vi "Tester_v01.vi"() -> ()   [LabVIEW 2015]
uses:
  <vilib>/LabVIEW Interface for Arduino/Type Defs/Pin Mode.ctl
  <vilib>/LabVIEW Interface for Arduino/LabVIEW Interface for Arduino.lvlib
panel:
  out "Test pass 2":string
  out "Welcome Message":string
  out "K4 voltage":dbl(knob) scale=0.0..5.0
  out "J16":dbl(knob) scale=0.0..5.0
  out "K3 voltage 2":dbl(knob) scale=0.0..5.0
  out "J6":dbl(knob) scale=0.0..5.0
  out "K2 voltage":dbl(knob) scale=0.0..5.0
  out "K1 voltage":dbl(knob) scale=0.0..5.0
  out "Tab Control":T1(tab)
  out "Please wait":string
  in  "Exit the program":bool
  in  "Start Test":bool
  in  "CONTINUE 2":bool
  out "Message Page 2":string
  in  "START page 3":bool
  out "Wire connection 3":string
  in  "NO LED ON":bool
  in  "YES LED ON":bool
  out "LED ON?":string
  out "Error message":string
  in  "STOP K1 LED ON":bool
  out "LED OFF?":string
  in  "YES LED OFF":bool
  in  "NO LED OFF":bool
  in  "STOP K1 LED OFF":bool
  out "Loading bar":string
  out "Progress Bar":u8(slide) scale=0.0..100.0
  in  "Stop K1":bool
  in  "STOP K2":bool
  in  "STOP K3":bool
  in  "STOP K4":bool
  in  "STOPJ6":bool
  in  "STOP J16":bool
  in  "STOP J4 error":bool
  out "Test pass":string
  in  "Complete":bool
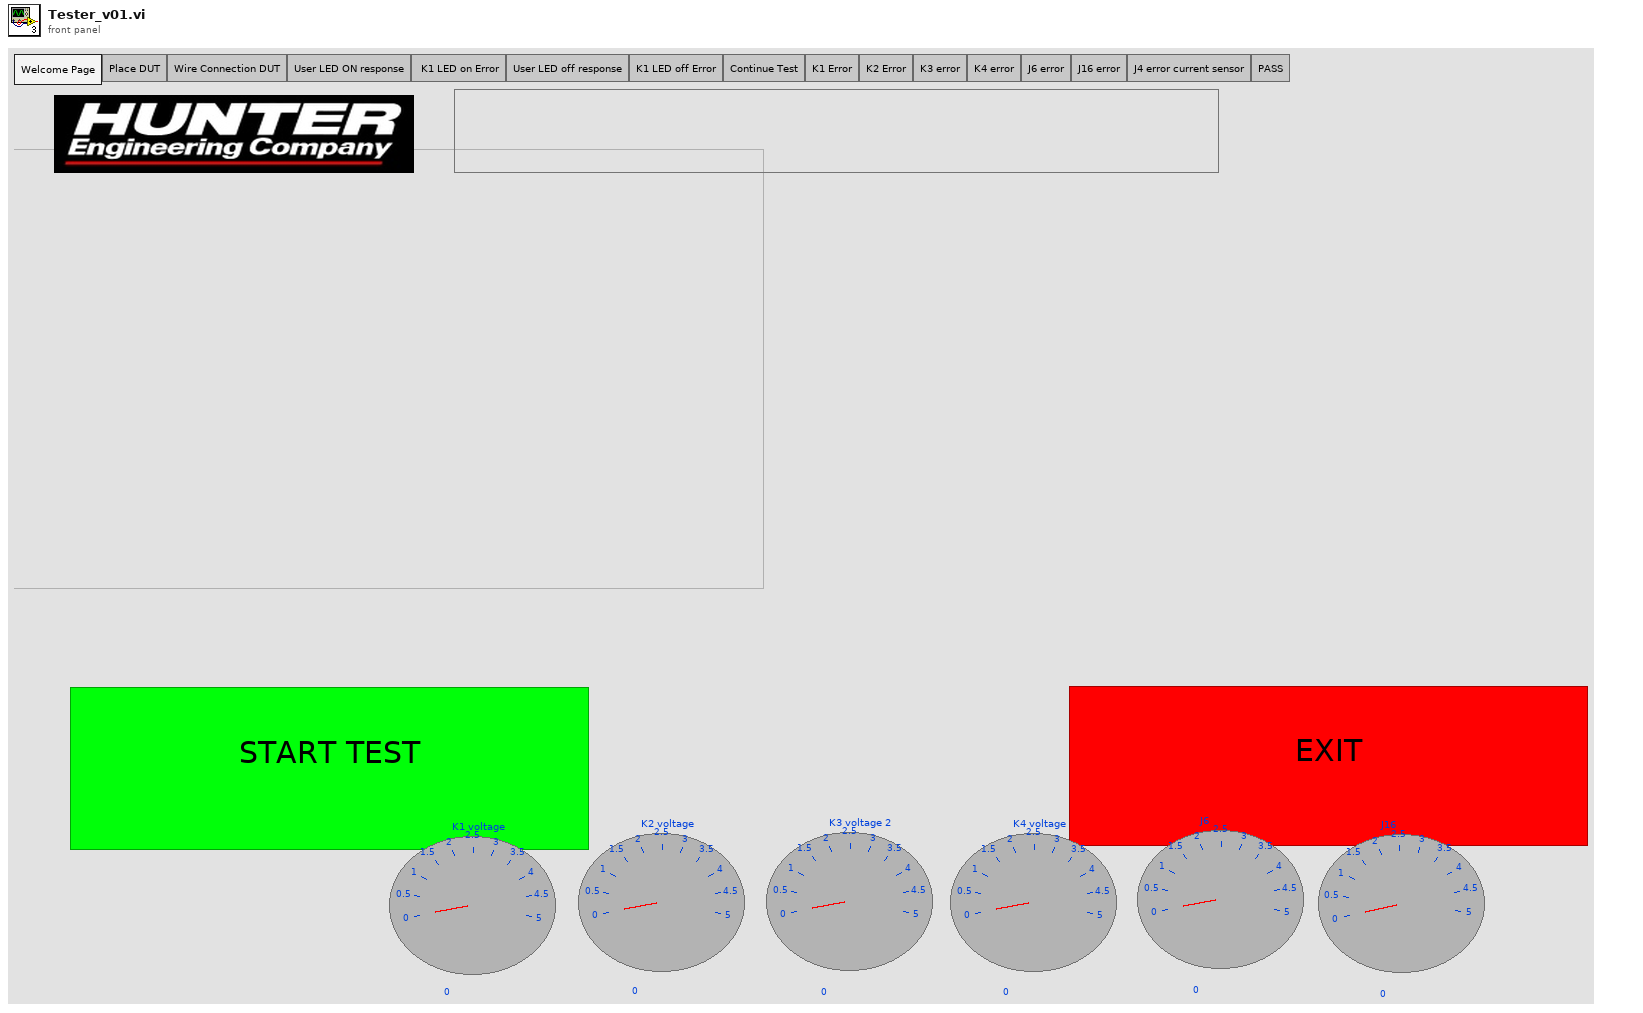
[diagram p1: front panel]
types:
  T1 = enum32{"Welcome Page", "Place DUT", "Wire Connection DUT", "User LED ON response", " K1 LED on Error", "User LED off response", "K1 LED off Error", "Continue Test", "K1 Error", "K2 Error", "K3 error", "K4 error", "J6 error", "J16 error", "J4 error current sensor", "PASS"}
  T2 = typedef "LabVIEW Interface for Arduino.lvlib/Pin Mode.ctl" = enum8{"Input", "Output"}
  T3 = enum8{"Enabled", "Disabled", "Disabled and Grayed Out"}
  T4 = typedef "LabVIEW Interface for Arduino.lvlib/Arduino Resource.ctl" = cluster{"VISA resource":refnum<visa-resource-name>, "Board Type":T5, "Connection Type":enum8{"USB / Serial"}, "Bytes Per Packet (15)":u8}
  T5 = typedef "LabVIEW Interface for Arduino.lvlib/Board Type.ctl" = enum16{"Uno", "Dimuelanove w/Atmega 328", "Mega 2560"}
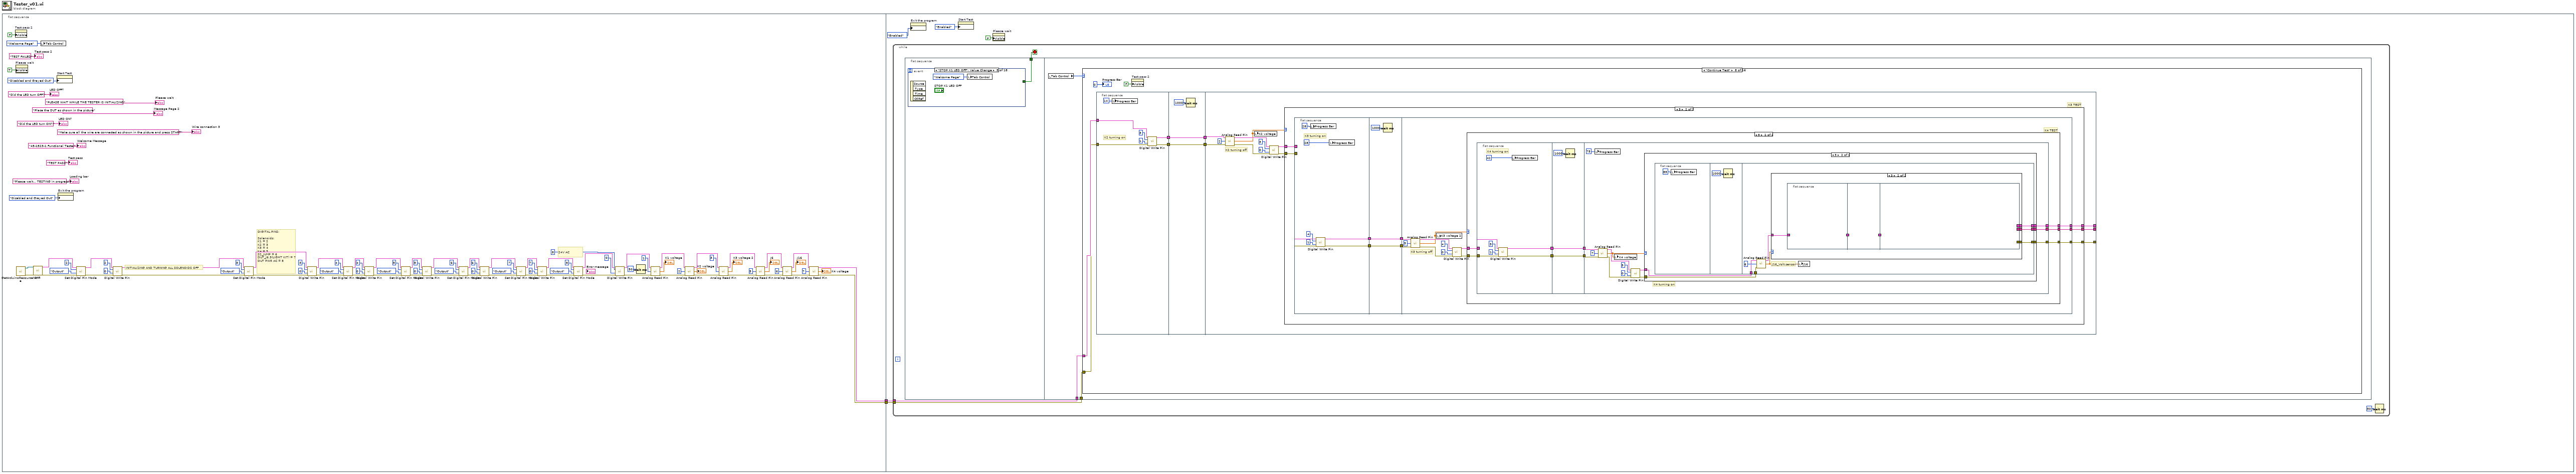
[diagram p0: block diagram]
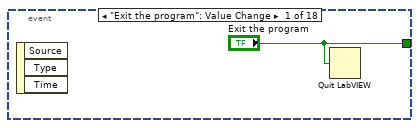
[diagram p2: hidden frame]
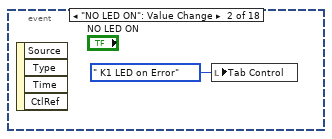
[diagram p3: hidden frame]
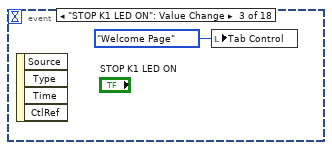
[diagram p4: hidden frame]
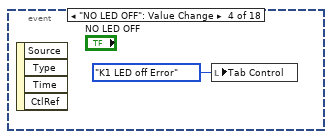
[diagram p5: hidden frame]
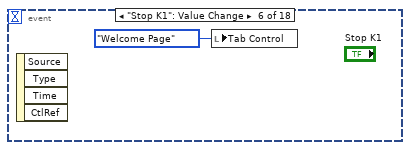
[diagram p6: hidden frame]
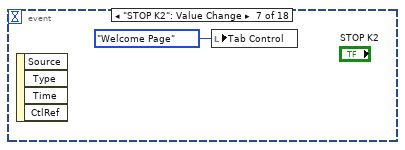
[diagram p7: hidden frame]
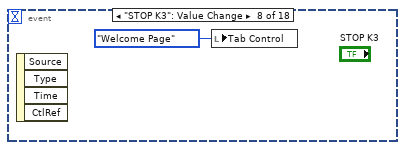
[diagram p8: hidden frame]
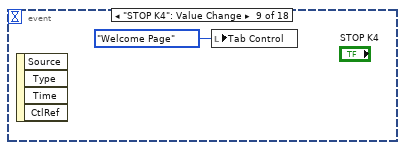
[diagram p9: hidden frame]
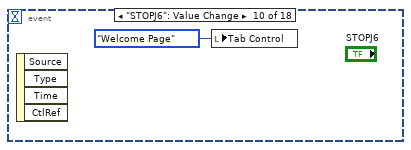
[diagram p10: hidden frame]
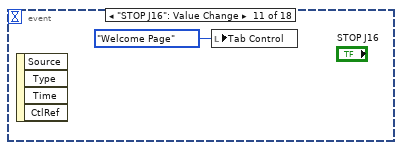
[diagram p11: hidden frame]
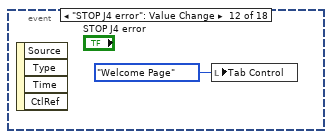
[diagram p12: hidden frame]
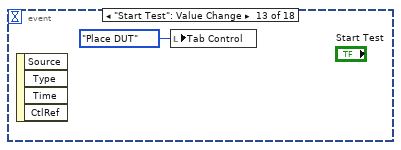
[diagram p13: hidden frame]
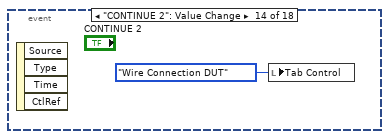
[diagram p14: hidden frame]
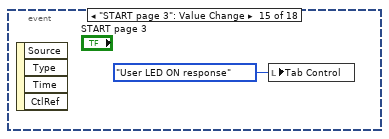
[diagram p15: hidden frame]
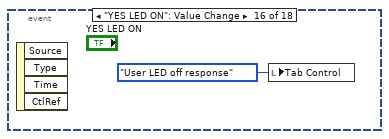
[diagram p16: hidden frame]
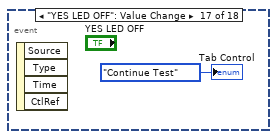
[diagram p17: hidden frame]
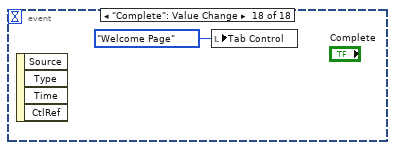
[diagram p18: hidden frame]
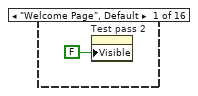
[diagram p19: hidden frame]
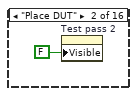
[diagram p20: hidden frame]
diagram:
  n1 = flat-sequence {
    tunnel: [w6] -> w2
    tunnel: [w5] -> w1
    tunnel: w2 -> [w106]
    tunnel: w1 -> [w105]
    frame #0 {
      # "24V AC"
      # "DIGITAL PINS:\n\nSolenoids:\nK1 = 2\nK2 = 3\nK3 = 4\nK4 = 5\nS2_JUMP = 6\nDUT_J6.3(LIGHT KIT) = 7\nDUT PWR AC = 8"
      # "INITIALIZING AND TURNING ALL SOLENOIDS OFF"
      n2 = property on="Test pass 2" class="Str"("Visible"=FALSE) -> ()  [unwired: 2 in, 2 out]
      n3 = property on="Please wait" class="Str"("Visible"=TRUE) -> ()  [unwired: 2 in, 2 out]
      n4 = call "GetArduinoResourceName.vi"() -> ("error out"=w39:errorcluster, "VISA resource name"=w40:refnum<visa-resource-name>)  [unwired: 10 in]
      n5 = call <vilib>:"Init.vi"("VISA resource"=w40, "error in"=w39) -> ("Arduino Resource"=w76:T4, "error out"=w75:errorcluster)  [unwired: 16 in]
      n6 = local write "Tab Control"(T1."Welcome Page" ("Tab Control")) -> ()
      n7 = property on="Start Test" class="Bool (strict)"("DisabledEnum"=T3."Disabled and Grayed Out" ("Disabled")) -> ()  [unwired: 2 in, 2 out]
      n8 = property on="Exit the program" class="Bool (strict)"("DisabledEnum"=T3."Disabled and Grayed Out" ("Disabled")) -> ()  [unwired: 2 in, 2 out]
      n9 = call <vilib>:"Set Digital Pin Mode.vi"("Arduino Resource"=w76, "Digital I/O Pin"=u8 2, "Pin Mode (Input)"=Pin_Mode."Output", "error in"=w75) -> ("Arduino Resource"=w96:T4, "error out"=w97:errorcluster)  [unwired: 10 in]
      n10 = call <vilib>:"Digital Write Pin.vi"("Arduino Resource"=w96, "Digital I/O Pin (0)"=u8 2 ("Digital I/O Pin"), "Value (0)"=u8 0, "error in"=w97) -> ("Arduino Resource"=w88:T4, "error out"=w87:errorcluster)  [unwired: 10 in]
      n11 = call <vilib>:"Set Digital Pin Mode.vi"("Arduino Resource"=w88, "Digital I/O Pin"=u8 3, "Pin Mode (Input)"=Pin_Mode."Output", "error in"=w87) -> ("Arduino Resource"=w91:T4, "error out"=w90:errorcluster)  [unwired: 10 in]
      n12 = call <vilib>:"Digital Write Pin.vi"("Arduino Resource"=w91, "Digital I/O Pin (0)"=u8 3 ("Digital I/O Pin"), "Value (0)"=u8 0, "error in"=w90) -> ("Arduino Resource"=w78:T4, "error out"=w77:errorcluster)  [unwired: 10 in]
      n13 = call <vilib>:"Set Digital Pin Mode.vi"("Arduino Resource"=w78, "Digital I/O Pin"=u8 4, "Pin Mode (Input)"=Pin_Mode."Output", "error in"=w77) -> ("Arduino Resource"=w42:T4, "error out"=w80:errorcluster)  [unwired: 10 in]
      n14 = call <vilib>:"Digital Write Pin.vi"("Arduino Resource"=w42, "Digital I/O Pin (0)"=u8 4 ("Digital I/O Pin"), "Value (0)"=u8 0, "error in"=w80) -> ("Arduino Resource"=w85:T4, "error out"=w86:errorcluster)  [unwired: 10 in]
      n15 = call <vilib>:"Set Digital Pin Mode.vi"("Arduino Resource"=w85, "Digital I/O Pin"=u8 5, "Pin Mode (Input)"=Pin_Mode."Output", "error in"=w86) -> ("Arduino Resource"=w36:T4, "error out"=w24:errorcluster)  [unwired: 10 in]
      n16 = call <vilib>:"Digital Write Pin.vi"("Arduino Resource"=w36, "Digital I/O Pin (0)"=u8 5 ("Digital I/O Pin"), "Value (0)"=u8 0, "error in"=w24) -> ("Arduino Resource"=w48:T4, "error out"=w47:errorcluster)  [unwired: 10 in]
      n17 = call <vilib>:"Set Digital Pin Mode.vi"("Arduino Resource"=w48, "Digital I/O Pin"=u8 6, "Pin Mode (Input)"=Pin_Mode."Output", "error in"=w47) -> ("Arduino Resource"=w55:T4, "error out"=w67:errorcluster)  [unwired: 10 in]
      n18 = call <vilib>:"Digital Write Pin.vi"("Arduino Resource"=w55, "Digital I/O Pin (0)"=u8 6 ("Digital I/O Pin"), "Value (0)"=u8 0, "error in"=w67) -> ("Arduino Resource"=w52:T4, "error out"=w51:errorcluster)  [unwired: 10 in]
      n19 = call <vilib>:"Set Digital Pin Mode.vi"("Arduino Resource"=w52, "Digital I/O Pin"=u8 7, "Pin Mode (Input)"=Pin_Mode."Output", "error in"=w51) -> ("Arduino Resource"=w54:T4, "error out"=w64:errorcluster)  [unwired: 10 in]
      n20 = call <vilib>:"Digital Write Pin.vi"("Arduino Resource"=w54, "Digital I/O Pin (0)"=u8 7 ("Digital I/O Pin"), "Value (0)"=u8 0, "error in"=w64) -> ("Arduino Resource"=w50:T4, "error out"=w49:errorcluster)  [unwired: 10 in]
      n21 = call <vilib>:"Set Digital Pin Mode.vi"("Arduino Resource"=w50, "Digital I/O Pin"=u8 8, "Pin Mode (Input)"=Pin_Mode."Output", "error in"=w49) -> ("Arduino Resource"=w53:T4, "error out"=w57:errorcluster)  [unwired: 10 in]
      n22 = call <vilib>:"Digital Write Pin.vi"("Arduino Resource"=w53, "Digital I/O Pin (0)"=u8 8 ("Digital I/O Pin"), "Value (0)"=u8 0, "error in"=w57) -> ("Arduino Resource"=w13:T4, "error out"=w14:errorcluster)  [unwired: 10 in]
      n23 = Wait (ms)(milliseconds to wait=u32 50) -> ()  [unwired: 1 out]
      n24 = call <vilib>:"Analog Read Pin.vi"("Arduino Resource"=w13, "Analog Input Pin (0)"=u8 1, "error in"=w14) -> ("Arduino Resource"=w4:T4, "Voltage"=→"K1 voltage":dbl, "error out"=w25:errorcluster)  [unwired: 10 in]
      n25 = call <vilib>:"Analog Read Pin.vi"("Arduino Resource"=w4, "Analog Input Pin (0)"=u8 2, "error in"=w25) -> ("Arduino Resource"=w3:T4, "Voltage"=→"K2 voltage":dbl, "error out"=w20:errorcluster)  [unwired: 10 in]
      n26 = call <vilib>:"Analog Read Pin.vi"("Arduino Resource"=w3, "Analog Input Pin (0)"=u8 3, "error in"=w20) -> ("Arduino Resource"=w23:T4, "Voltage"=→"K3 voltage 2":dbl, "error out"=w21:errorcluster)  [unwired: 10 in]
      n27 = call <vilib>:"Analog Read Pin.vi"("Arduino Resource"=w23, "Analog Input Pin (0)"=u8 5, "error in"=w21) -> ("Arduino Resource"=w22:T4, "Voltage"=→"J6":dbl, "error out"=w19:errorcluster)  [unwired: 10 in]
      n28 = call <vilib>:"Analog Read Pin.vi"("Arduino Resource"=w22, "Analog Input Pin (0)"=u8 6, "error in"=w19) -> ("Arduino Resource"=w16:T4, "Voltage"=→"J16":dbl, "error out"=w17:errorcluster)  [unwired: 10 in]
      n29 = call <vilib>:"Analog Read Pin.vi"("Arduino Resource"=w16, "Analog Input Pin (0)"=u8 7, "error in"=w17) -> ("Arduino Resource"=w6:T4, "Voltage"=→"K4 voltage":dbl, "error out"=w5:errorcluster)  [unwired: 10 in]
      "Welcome Message" <- "45-1523-1 Functional Tester"
      "Message Page 2" <- "Place the DUT as shown in the picture"
      "Wire connection 3" <- "Make sure all the wire are connected as shown in the picture and press START" ("Wire connection 3")
      "LED ON?" <- "Did the LED turn ON?!" ("LED ON?")
      "LED OFF?" <- "Did the LED turn OFF?" ("LED OFF?")
      "Loading bar" <- "Please wait... TESTING in progress" ("Loading bar")
      "Test pass" <- "TEST PASS" ("Test pass")
      "Please wait" <- "PLEASE WAIT WHILE THE TESTER IS INITIALIZING" ("Please wait")
      "Test pass 2" <- "TEST FAILED" ("Test pass 2")
    }
    frame #1 {
      n30 = while {
        tunnel: w106 -> [w109]
        tunnel: w105 -> [w108]
        stop <- w107 stop-if-true
        n31 = flat-sequence {
          tunnel: [w111] -> w107
          tunnel: w109 -> [w132]
          tunnel: w108 -> [w131]
          frame #0 {
            n32 = event shown="[4] \"STOP K1 LED OFF\": Value Change" {
              selector: _ -> [_ _ _ _ _ _ _ _ _ _ _ _ _ _ _ _ _ _]
              dyn-events: _ -> [_ _ _ _ _ _ _ _ _ _ _ _ _ _ _ _ _ _]
              timeout: _ -> [_ _ _ _ _ _ _ _ _ _ _ _ _ _ _ _ _ _]
              tunnel: ["Exit the program" _ _ _ _ _ _ _ _ _ _ _ _ _ _ _ _ _] -> w111
              event "Exit the program": Value Change {
                n33 = event-data() -> ()  [unwired: 1 in, 3 out]
                n34 = Quit LabVIEW(quit? (T)="Exit the program") -> ()
              }
              event "NO LED ON": Value Change {
                n35 = event-data() -> ()  [unwired: 1 in, 4 out]
                n36 = local write "Tab Control"(T1." K1 LED on Error" ("Tab Control")) -> ()
              }
              event "STOP K1 LED ON": Value Change {
                n37 = event-data() -> ()  [unwired: 1 in, 4 out]
                n38 = local write "Tab Control"(T1."Welcome Page" ("Tab Control")) -> ()
              }
              event "NO LED OFF": Value Change {
                n39 = event-data() -> ()  [unwired: 1 in, 4 out]
                n40 = local write "Tab Control"(T1."K1 LED off Error" ("Tab Control")) -> ()
              }
              event "STOP K1 LED OFF": Value Change {
                n41 = event-data() -> ()  [unwired: 1 in, 4 out]
                n42 = local write "Tab Control"(T1."Welcome Page" ("Tab Control")) -> ()
              }
              event "Stop K1": Value Change {
                n43 = event-data() -> ()  [unwired: 1 in, 4 out]
                n44 = local write "Tab Control"(T1."Welcome Page" ("Tab Control")) -> ()
              }
              event "STOP K2": Value Change {
                n45 = event-data() -> ()  [unwired: 1 in, 4 out]
                n46 = local write "Tab Control"(T1."Welcome Page" ("Tab Control")) -> ()
              }
              event "STOP K3": Value Change {
                n47 = event-data() -> ()  [unwired: 1 in, 4 out]
                n48 = local write "Tab Control"(T1."Welcome Page" ("Tab Control")) -> ()
              }
              event "STOP K4": Value Change {
                n49 = event-data() -> ()  [unwired: 1 in, 4 out]
                n50 = local write "Tab Control"(T1."Welcome Page" ("Tab Control")) -> ()
              }
              event "STOPJ6": Value Change {
                n51 = event-data() -> ()  [unwired: 1 in, 4 out]
                n52 = local write "Tab Control"(T1."Welcome Page" ("Tab Control")) -> ()
              }
              event "STOP J16": Value Change {
                n53 = event-data() -> ()  [unwired: 1 in, 4 out]
                n54 = local write "Tab Control"(T1."Welcome Page" ("Tab Control")) -> ()
              }
              event "STOP J4 error": Value Change {
                n55 = event-data() -> ()  [unwired: 1 in, 4 out]
                n56 = local write "Tab Control"(T1."Welcome Page" ("Tab Control")) -> ()
              }
              event "Start Test": Value Change {
                n57 = event-data() -> ()  [unwired: 1 in, 4 out]
                n58 = local write "Tab Control"(T1."Place DUT" ("Tab Control")) -> ()
              }
              event "CONTINUE 2": Value Change {
                n59 = event-data() -> ()  [unwired: 1 in, 4 out]
                n60 = local write "Tab Control"(T1."Wire Connection DUT" ("Tab Control")) -> ()
              }
              event "START page 3": Value Change {
                n61 = event-data() -> ()  [unwired: 1 in, 4 out]
                n62 = local write "Tab Control"(T1."User LED ON response" ("Tab Control")) -> ()
              }
              event "YES LED ON": Value Change {
                n63 = event-data() -> ()  [unwired: 1 in, 4 out]
                n64 = local write "Tab Control"(T1."User LED off response" ("Tab Control")) -> ()
              }
              event "YES LED OFF": Value Change {
                n65 = event-data() -> ()  [unwired: 1 in, 4 out]
                "Tab Control" <- T1."Continue Test" ("Tab Control")
              }
              event "Complete": Value Change {
                n66 = event-data() -> ()  [unwired: 1 in, 4 out]
                n67 = local write "Tab Control"(T1."Welcome Page" ("Tab Control")) -> ()
              }
            }
          }
          frame #1 {
            n68 = local read "Tab Control"() -> (w130:T1)
            n69 = case shown="\"Continue Test\"" w130 {
              tunnel: w132 -> [_ _ _ w149 _ w186 _ w210 _ _ _ _ _ _ _ _]
              tunnel: w131 -> [_ _ _ w148 _ w185 _ w209 _ _ _ _ _ _ _ _]
              frame "Welcome Page", Default {
                n70 = property on="Test pass 2" class="Str"("Visible"=FALSE) -> ()  [unwired: 2 in, 2 out]
              }
              frame "Place DUT" {
                n71 = property on="Test pass 2" class="Str"("Visible"=FALSE) -> ()  [unwired: 2 in, 2 out]
              }
              frame "Wire Connection DUT" {
                n72 = property on="Test pass 2" class="Str"("Visible"=FALSE) -> ()  [unwired: 2 in, 2 out]
              }
              frame "User LED ON response" {
                n73 = flat-sequence {
                  tunnel: w149 -> [w153]
                  tunnel: w148 -> [w152]
                  tunnel: [w151] -> w139
                  tunnel: [w150] -> w137
                  tunnel: w139 -> [w158]
                  tunnel: [w158] -> w138
                  tunnel: w137 -> [w157]
                  tunnel: [w157] -> w136
                  tunnel: w138 -> [w163]
                  tunnel: [w162] -> w141
                  tunnel: [w161] -> w140
                  tunnel: w136 -> [w160]
                  tunnel: [w166] -> w147
                  tunnel: [w165] -> w146
                  tunnel: w141 -> [w166]
                  tunnel: w140 -> [w165]
                  tunnel: w147 -> [w172]
                  tunnel: w146 -> [w171]
                  tunnel: [w170] -> w144
                  tunnel: [w169] -> w143
                  tunnel: [w168] -> w142
                  tunnel: w144 -> [w177]
                  tunnel: w143 -> [w176]
                  tunnel: w142 -> [w178]
                  frame #0 {
                    n74 = call <vilib>:"Digital Write Pin.vi"("Arduino Resource"=w153, "Digital I/O Pin (0)"=u8 8, "Value (0)"=u8 1, "error in"=w152) -> ("Arduino Resource"=w150:T4, "error out"=w151:errorcluster)  [unwired: 10 in]
                  }
                  frame #1 {
                    n75 = Wait (ms)(milliseconds to wait=u32 1000) -> ()  [unwired: 1 out]
                  }
                  frame #2 {
                    n76 = call <vilib>:"Digital Write Pin.vi"("Arduino Resource"=w160, "Digital I/O Pin (0)"=u8 2, "Value (0)"=u8 1, "error in"=w163) -> ("Arduino Resource"=w162:T4, "error out"=w161:errorcluster)  [unwired: 10 in]
                  }
                  frame #3 {
                    n77 = Wait (ms)(milliseconds to wait=u32 1000) -> ()  [unwired: 1 out]
                  }
                  frame #4 {
                    n78 = call <vilib>:"Analog Read Pin.vi"("Arduino Resource"=w172, "Analog Input Pin (0)"=u8 1, "error in"=w171) -> ("Arduino Resource"=w168:T4, "Voltage"=w169:dbl, "error out"=w170:errorcluster)  [unwired: 10 in]
                  }
                  frame #5 {
                    n79 = call <vilib>:"Digital Write Pin.vi"("Arduino Resource"=w178, "Digital I/O Pin (0)"=u8 2, "Value (0)"=u8 0, "error in"=w177) -> ()  [unwired: 10 in, 2 out]
                    n80 = local write "K1 voltage"(w176) -> ()
                  }
                }
                n81 = property on="Test pass 2" class="Str"("Visible"=FALSE) -> ()  [unwired: 2 in, 2 out]
              }
              frame " K1 LED on Error" {
                n82 = property on="Test pass 2" class="Str"("Visible"=TRUE) -> ()  [unwired: 2 in, 2 out]
              }
              frame "User LED off response" {
                n83 = flat-sequence {
                  tunnel: w186 -> [w194]
                  tunnel: w185 -> [w193]
                  tunnel: [w189] -> w183
                  tunnel: [w188] -> w181
                  tunnel: [w198] -> w184
                  tunnel: w183 -> [w198]
                  tunnel: [w197] -> w182
                  tunnel: w181 -> [w197]
                  tunnel: w184 -> [w202]
                  tunnel: w182 -> [w201]
                  frame #0 {
                    n84 = call <vilib>:"Digital Write Pin.vi"("Arduino Resource"=w194, "Digital I/O Pin (0)"=u8 7, "Value (0)"=u8 1, "error in"=w193) -> ("Arduino Resource"=w191:T4, "error out"=w190:errorcluster)  [unwired: 10 in]
                    n85 = call <vilib>:"Digital Write Pin.vi"("Arduino Resource"=w191, "Digital I/O Pin (0)"=u8 6, "Value (0)"=u8 1, "error in"=w190) -> ("Arduino Resource"=w189:T4, "error out"=w188:errorcluster)  [unwired: 10 in]
                  }
                  frame #1 {
                    n86 = Wait (ms)(milliseconds to wait=u32 250) -> ()  [unwired: 1 out]
                  }
                  frame #2 {
                    n87 = call <vilib>:"Digital Write Pin.vi"("Arduino Resource"=w202, "Digital I/O Pin (0)"=u8 7, "Value (0)"=u8 0, "error in"=w201) -> ("Arduino Resource"=w206:T4, "error out"=w207:errorcluster)  [unwired: 10 in]
                    n88 = call <vilib>:"Digital Write Pin.vi"("Arduino Resource"=w206, "Digital I/O Pin (0)"=u8 6, "Value (0)"=u8 0, "error in"=w207) -> ()  [unwired: 10 in, 2 out]
                  }
                }
                n89 = property on="Test pass 2" class="Str"("Visible"=FALSE) -> ()  [unwired: 2 in, 2 out]
              }
              frame "K1 LED off Error" {
                n90 = property on="Test pass 2" class="Str"("Visible"=TRUE) -> ()  [unwired: 2 in, 2 out]
              }
              frame "Continue Test" {
                n91 = flat-sequence {
                  tunnel: [w221] -> w215
                  tunnel: [w220] -> w214
                  tunnel: w210 -> [w218]
                  tunnel: w209 -> [w217]
                  tunnel: w215 -> [w224]
                  tunnel: [w225] -> w213
                  tunnel: w214 -> [w225]
                  tunnel: [w224] -> w212
                  tunnel: w213 -> [w238]
                  tunnel: w212 -> [w237]
                  tunnel: [w230] -> _
                  tunnel: [w228] -> _
                  tunnel: [w227] -> _
                  frame #0 {
                    # "K2 turning on"
                    n92 = local write "Progress Bar"(u8 14 ("Progress Bar")) -> ()
                    n93 = call <vilib>:"Digital Write Pin.vi"("Arduino Resource"=w218, "Digital I/O Pin (0)"=u8 3, "Value (0)"=u8 1, "error in"=w217) -> ("Arduino Resource"=w221:T4, "error out"=w220:errorcluster)  [unwired: 10 in]
                  }
                  frame #1 {
                    n94 = Wait (ms)(milliseconds to wait=u32 1000) -> ()  [unwired: 1 out]
                  }
                  frame #2 {
                    # "K3 TEST"
                    # "K2 turning off"
                    n95 = call <vilib>:"Analog Read Pin.vi"("Arduino Resource"=w237, "Analog Input Pin (0)"=u8 2, "error in"=w238) -> ("Arduino Resource"=w236:T4, "Voltage"=w229:dbl, "error out"=w235:errorcluster)  [unwired: 10 in]
                    n96 = local write "K2 voltage"(w229) -> ()
                    n97 = call <vilib>:"Digital Write Pin.vi"("Arduino Resource"=w236, "Digital I/O Pin (0)"=u8 3, "Value (0)"=u8 0, "error in"=w235) -> ("Arduino Resource"=w232:T4, "error out"=w231:errorcluster)  [unwired: 10 in]
                    n98 = case shown="5" w229 {
                      tunnel: w231 -> [_ w249]
                      tunnel: w232 -> [_ w248]
                      tunnel: [_ w244] -> w230
                      tunnel: [_ w243] -> w228
                      tunnel: [_ w242] -> w227
                      frame 0, Default {
                        n99 = property on="Test pass 2" class="Str"("Visible"=TRUE) -> ()  [unwired: 2 in, 2 out]
                        n100 = local write "Tab Control"(T1."K2 Error" ("Tab Control")) -> ()
                      }
                      frame 5 {
                        n101 = flat-sequence {
                          tunnel: [w256] -> w250
                          tunnel: w249 -> [w255]
                          tunnel: w248 -> [w254]
                          tunnel: [w253] -> w247
                          tunnel: w250 -> [w259]
                          tunnel: w247 -> [w260]
                          tunnel: [w260] -> w246
                          tunnel: [w259] -> w245
                          tunnel: w246 -> [w273]
                          tunnel: w245 -> [w272]
                          tunnel: [w266] -> w244
                          tunnel: [w264] -> w243
                          tunnel: [w263] -> w242
                          frame #0 {
                            # "K3 turning on"
                            n102 = local write "Progress Bar"(u8 28 ("Progress Bar")) -> ()
                            n103 = call <vilib>:"Digital Write Pin.vi"("Arduino Resource"=w254, "Digital I/O Pin (0)"=u8 4, "Value (0)"=u8 1, "error in"=w255) -> ("Arduino Resource"=w253:T4, "error out"=w256:errorcluster)  [unwired: 10 in]
                            n104 = local write "Progress Bar"(u8 28 ("Progress Bar")) -> ()
                          }
                          frame #1 {
                            n105 = Wait (ms)(milliseconds to wait=u32 1000) -> ()  [unwired: 1 out]
                          }
                          frame #2 {
                            # "K4 TEST"
                            # "K3 turning off"
                            n106 = call <vilib>:"Analog Read Pin.vi"("Arduino Resource"=w273, "Analog Input Pin (0)"=u8 3, "error in"=w272) -> ("Arduino Resource"=w262:T4, "Voltage"=w265:dbl, "error out"=w271:errorcluster)  [unwired: 10 in]
                            n107 = local write "K3 voltage 2"(w265) -> ()
                            n108 = call <vilib>:"Digital Write Pin.vi"("Arduino Resource"=w262, "Digital I/O Pin (0)"=u8 4, "Value (0)"=u8 0, "error in"=w271) -> ("Arduino Resource"=w270:T4, "error out"=w269:errorcluster)  [unwired: 10 in]
                            n109 = case shown="5" w265 {
                              tunnel: w270 -> [_ w281]
                              tunnel: w269 -> [_ w280]
                              tunnel: [_ w279] -> w266
                              tunnel: [_ w278] -> w264
                              tunnel: [_ w277] -> w263
                              frame 0, Default {
                                n110 = property on="Test pass 2" class="Str"("Visible"=TRUE) -> ()  [unwired: 2 in, 2 out]
                                n111 = local write "Tab Control"(T1."K3 error" ("Tab Control")) -> ()
                              }
                              frame 5 {
                                n112 = flat-sequence {
                                tunnel: [w290] -> w285
                                tunnel: [w289] -> w284
                                tunnel: w281 -> [w287]
                                tunnel: w280 -> [w286]
                                tunnel: w285 -> [w293]
                                tunnel: [w294] -> w283
                                tunnel: w284 -> [w294]
                                tunnel: [w293] -> w282
                                tunnel: w283 -> [w306]
                                tunnel: w282 -> [w307]
                                tunnel: [w300] -> w279
                                tunnel: [w298] -> w278
                                tunnel: [w297] -> w277
                                frame #0 {
                                # "K4 turning on"
                                n113 = call <vilib>:"Digital Write Pin.vi"("Arduino Resource"=w287, "Digital I/O Pin (0)"=u8 5, "Value (0)"=u8 1, "error in"=w286) -> ("Arduino Resource"=w290:T4, "error out"=w289:errorcluster)  [unwired: 10 in]
                                n114 = local write "Progress Bar"(u8 42 ("Progress Bar")) -> ()
                                }
                                frame #1 {
                                n115 = Wait (ms)(milliseconds to wait=u32 1000) -> ()  [unwired: 1 out]
                                }
                                frame #2 {
                                # "K4 turning on"
                                n116 = local write "Progress Bar"(u8 75 ("Progress Bar")) -> ()
                                n117 = call <vilib>:"Analog Read Pin.vi"("Arduino Resource"=w307, "Analog Input Pin (0)"=u8 7, "error in"=w306) -> ("Arduino Resource"=w296:T4, "Voltage"=w299:dbl, "error out"=w303:errorcluster)  [unwired: 10 in]
                                n118 = local write "K4 voltage"(w299) -> ()
                                n119 = call <vilib>:"Digital Write Pin.vi"("Arduino Resource"=w296, "Digital I/O Pin (0)"=u8 5, "Value (0)"=u8 0, "error in"=w303) -> ("Arduino Resource"=w302:T4, "error out"=w301:errorcluster)  [unwired: 10 in]
                                n120 = case shown="3" w299 {
                                tunnel: w302 -> [_ w316]
                                tunnel: w301 -> [_ w315]
                                tunnel: [_ w314] -> w300
                                tunnel: [_ w313] -> w298
                                tunnel: [_ w312] -> w297
                                frame 0, Default {
                                n121 = property on="Test pass 2" class="Str"("Visible"=TRUE) -> ()  [unwired: 2 in, 2 out]
                                n122 = local write "Tab Control"(T1."K4 error" ("Tab Control")) -> ()
                                }
                                frame 3 {
                                n123 = flat-sequence {
                                tunnel: w316 -> [w325]
                                tunnel: w315 -> [w324]
                                tunnel: [w323] -> w314
                                tunnel: [w320] -> w313
                                tunnel: [w319] -> w312
                                frame #0 {
                                n124 = local write "Progress Bar"(u8 85 ("Progress Bar")) -> ()
                                }
                                frame #1 {
                                n125 = Wait (ms)(milliseconds to wait=u32 1000) -> ()  [unwired: 1 out]
                                }
                                frame #2 {
                                # "J16_Volt sensor"
                                n126 = call <vilib>:"Analog Read Pin.vi"("Arduino Resource"=w325, "Analog Input Pin (0)"=u8 6, "error in"=w324) -> ("Arduino Resource"=w321:T4, "Voltage"=w322:dbl)  [unwired: 10 in, 1 out]
                                n127 = case shown="3" w322 {
                                tunnel: [_ w331] -> w323
                                tunnel: w321 -> [_ w332]
                                tunnel: [_ w330] -> w320
                                tunnel: [_ w329] -> w319
                                frame 0, Default {
                                n128 = property on="Test pass 2" class="Str"("Visible"=TRUE) -> ()  [unwired: 2 in, 2 out]
                                n129 = local write "Tab Control"(T1."J16 error" ("Tab Control")) -> ()
                                }
                                frame 3 {
                                n130 = flat-sequence {
                                tunnel: [w335] -> w333
                                tunnel: w332 -> [w335]
                                tunnel: [w337] -> w334
                                tunnel: w333 -> [w337]
                                tunnel: [w343] -> w330
                                tunnel: [w342] -> w329
                                tunnel: [w341] -> w331
                                tunnel: w334 -> [w339]
                                frame #0 {
                                n131 = local write "Progress Bar"(u8 85 ("Progress Bar")) -> ()
                                }
                                frame #1 {
                                n132 = Wait (ms)(milliseconds to wait=u32 1000) -> ()  [unwired: 1 out]
                                }
                                frame #2 {
                                # "J6_Volt sensor"
                                n133 = call <vilib>:"Analog Read Pin.vi"("Arduino Resource"=w339, "Analog Input Pin (0)"=u8 5) -> ("Arduino Resource"=w343:T4, "Voltage"=w340:dbl, "error out"=w342:errorcluster)  [unwired: 11 in]
                                n134 = local write "J6"(w340) -> ()
                                n135 = case shown="0, Default" w340 {
                                tunnel: ["not completed" "completed"] -> w341
                                frame 0, Default {
                                n136 = property on="Test pass 2" class="Str"("Visible"=TRUE) -> ()  [unwired: 2 in, 2 out]
                                n137 = local write "Tab Control"(T1."J6 error" ("Tab Control")) -> ()
                                }
                                frame 3 {
                                n138 = local write "Tab Control"(T1."PASS" ("Tab Control")) -> ()
                                }
                                }
                                }
                                }
                                }
                                }
                                n139 = local write "J16"(w322) -> ()
                                }
                                }
                                }
                                }
                                }
                                }
                              }
                            }
                          }
                        }
                      }
                    }
                  }
                }
                n140 = property on="Test pass 2" class="Str"("Visible"=FALSE) -> ()  [unwired: 2 in, 2 out]
                "Progress Bar" <- u8 0 ("Progress Bar")
              }
              frame "K1 Error" {
              }
              frame "K2 Error" {
                n141 = property on="Test pass 2" class="Str"("Visible"=TRUE) -> ()  [unwired: 2 in, 2 out]
              }
              frame "K3 error" {
                n142 = property on="Test pass 2" class="Str"("Visible"=TRUE) -> ()  [unwired: 2 in, 2 out]
              }
              frame "K4 error" {
                n143 = property on="Test pass 2" class="Str"("Visible"=TRUE) -> ()  [unwired: 2 in, 2 out]
              }
              frame "J6 error" {
                n144 = property on="Test pass 2" class="Str"("Visible"=TRUE) -> ()  [unwired: 2 in, 2 out]
              }
              frame "J16 error" {
                n145 = property on="Test pass 2" class="Str"("Visible"=TRUE) -> ()  [unwired: 2 in, 2 out]
              }
              frame "J4 error current sensor" {
                n146 = property on="Test pass 2" class="Str"("Visible"=TRUE) -> ()  [unwired: 2 in, 2 out]
              }
              frame "PASS" {
                n147 = property on="Test pass 2" class="Str"("Visible"=FALSE) -> ()  [unwired: 2 in, 2 out]
              }
            }
          }
        }
        n148 = Wait (ms)(milliseconds to wait=u32 50) -> ()  [unwired: 1 out]
      }
      n149 = property on="Exit the program" class="Bool (strict)"("DisabledEnum"=T3."Enabled" ("Disabled")) -> ()  [unwired: 2 in, 2 out]
      n150 = property on="Start Test" class="Bool (strict)"("DisabledEnum"=T3."Enabled" ("Disabled")) -> ()  [unwired: 2 in, 2 out]
      n151 = property on="Please wait" class="Str"("Visible"=FALSE) -> ()  [unwired: 2 in, 2 out]
    }
  }
